vi "Multi-Record Acquisition with Queues.vi"() -> ()   [LabVIEW 2011]
uses:
  <vilib>/userDefined/High Color/nirio_resource_hc.ctl
  <vilib>/FPGAPlugInAG/PXIe-7965R/niLvFpga_Open_PXIe-7965R.vi
  <vilib>/rvi/interface/common/dynamic/niFpgaDynamicAddResources.vi
  <vilib>/FPGAPlugInAG/Dynamic/niLvFpga_Download_Dynamic.vi
  <vilib>/FPGAPlugInAG/Dynamic/niLvFpga_Run_Dynamic.vi
  <vilib>/Utility/error.llb/Error Cluster From Error Code.vi
  <vilib>/rvi/errors/niLvFpgaAdjustHostInterfaceError.vi
  <vilib>/FPGAPlugInAG/Dynamic/niLvFpga_Close_Dynamic.vi
  <vilib>/rvi/interface/nirviOpenFPGA/nirviOpenFPGA.xnode
  <userlib>/Fast OCT/Debug/Version 1/FPGA Bitfiles/Current/Acquire 2 channel data with DRAM (Multi-Record).lvbitx
  <vilib>/rvi/interface/nirviMethod/nirviMethod.xnode
  <vilib>/rvi/interface/nirviReadWriteControl/nirviReadWriteControl.xnode
  <vilib>/rvi/interface/nirviCloseFPGA/nirviCloseFPGA.xnode
  <userlib>/FlexRIO Host Library/FlexRIO Host Library (User).lvlib
  <vilib>/rvi/interface/Simulation/niFpgaSimulationCallBeginRW.vi
  NiFpgaLv.dll
panel:
  out "Consumer Stopped":bool
  out "Producer Stopped?":bool
  out "# elements in queue":i32
  out "Host FIFO Timed Out?":bool
  out "Buffer Timed Out?":bool
  out "Records Done":u32=500
  out "Elements Remaining":u32
  out "Iterations":i32=4
  in  "Display Raw Data?":bool=TRUE
  out "Channel Data":dbl[][](graph)
  out "Processing Time":u32=2246 format="%.0f ms"
  out "B-Scan Data":dbl[][](graph)
  in  "Device Name":T1="RIO0"
  in  "Stop":bool
  in  "Trigger Type":T2(ring)=enum."External Digital Trigger"
  in  "Record Count":u32=500
  in  "Pre Trig":u32=2
  in  "Post Trig":u32=1625
  out "error out":errorcluster
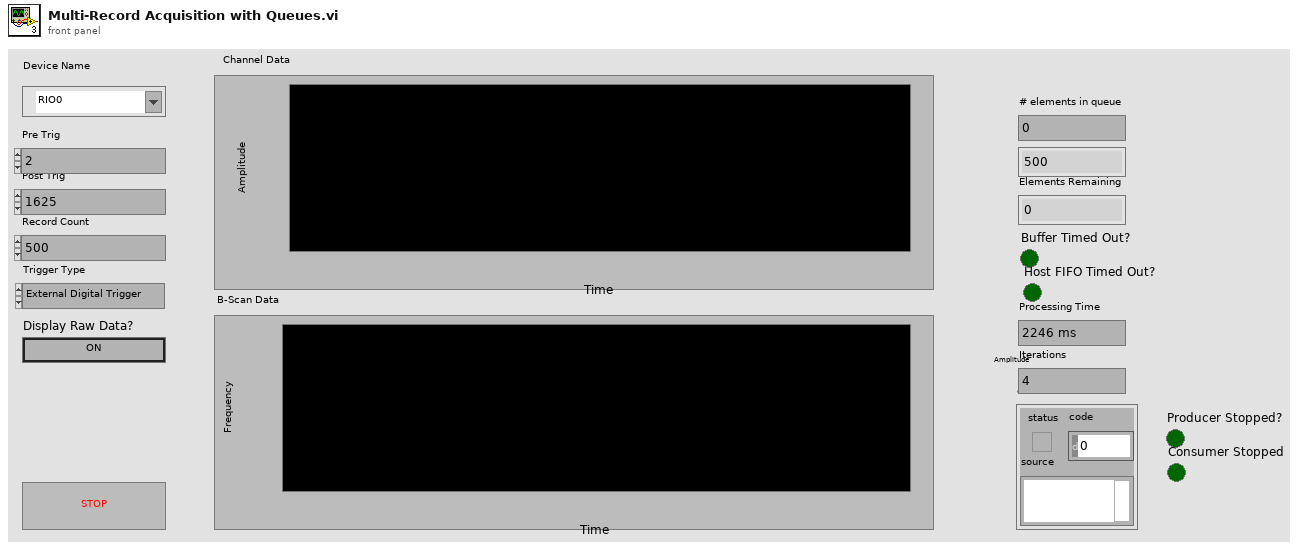
[diagram p1: front panel]
types:
  T1 = typedef "nirio_resource_hc.ctl" = tag
  T2 = enum8{"Immediate Trigger", "Software Trigger", "External Digital Trigger", "Analog Trigger"}
  T3 = cluster{"Load Record Parameters?":bool, "Pre Trigger Samples":u32, "Post Trigger Samples":u32, "Trigger Hold Off":u32, "Record Count":u32}
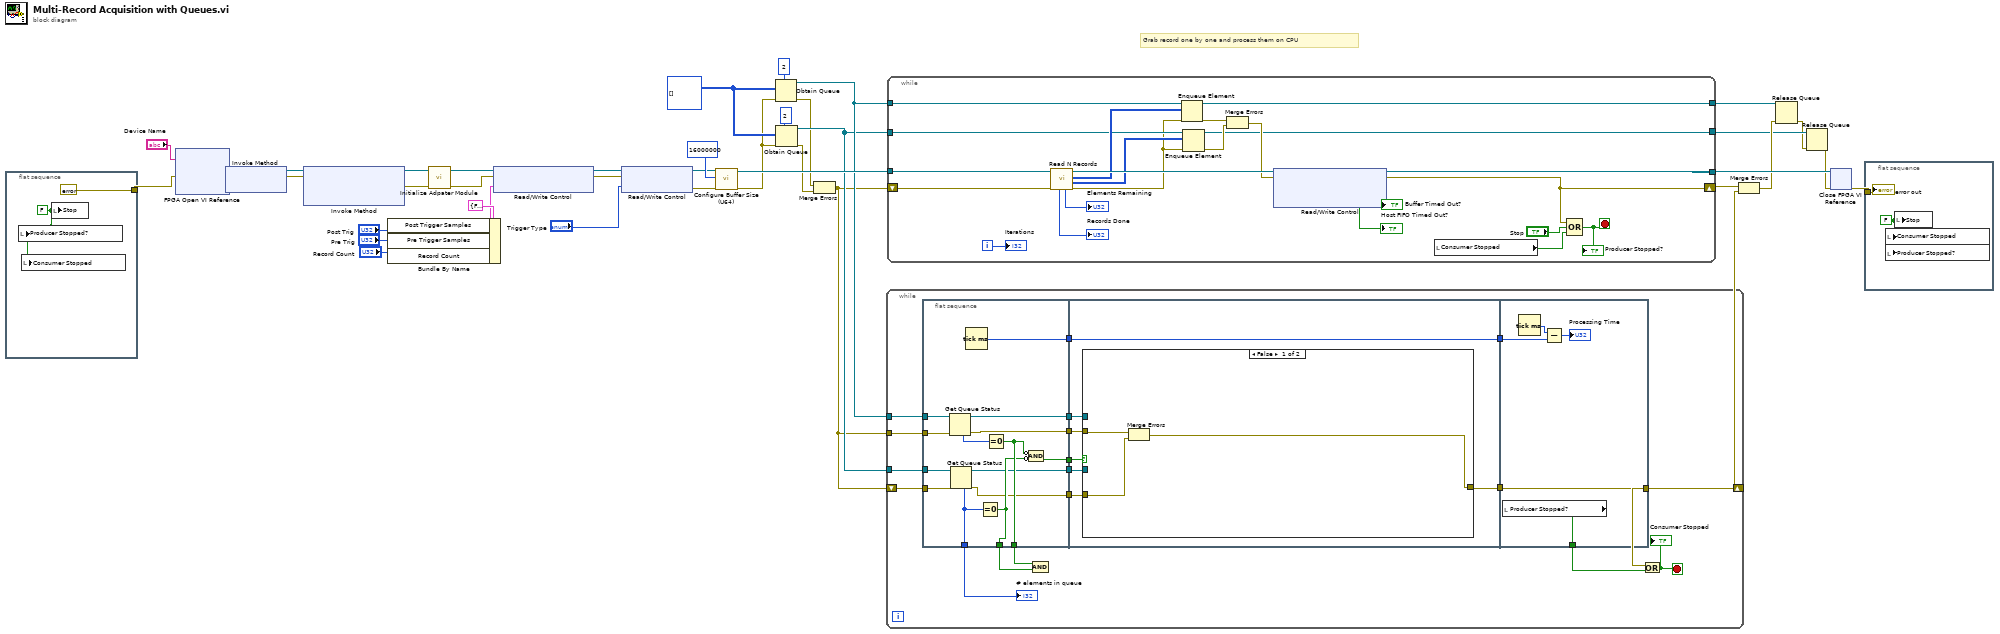
[diagram p0: block diagram]
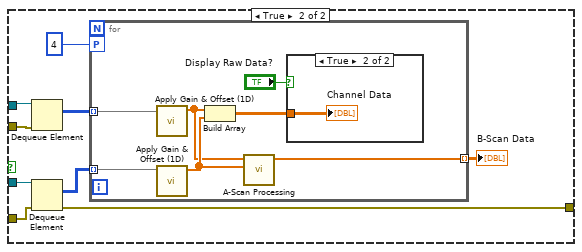
[diagram p2: hidden frame]
diagram:
  w16 = i16[][] [] ("Channel 1 Records")
  # "Grab record one by one and process them on CPU"
  n1 = flat-sequence {
    tunnel: [errorcluster {"status"=FALSE, "code"=0, "source"=""} ("error in")] -> w8
    frame #0 {
      w41 = FALSE ("Stop")
      n2 = local write "Producer Stopped?"(w41) -> ()
      n3 = local write "Consumer Stopped"(w41) -> ()
      n4 = local write "Stop"(w41) -> ()
    }
  }
  n5 = xnode "FPGA Open VI Reference"("error in"=w8, "resource name"="Device Name") -> ("FPGA VI Reference Out"=w22:refnum<k20>, "error out"=w23:errorcluster)
  n6 = xnode "Invoke Method"("FPGA VI Reference In"=w22, "error in"=w23) -> ("FPGA VI Reference Out"=w25:refnum<k20>, "error out"=w24:errorcluster)
  n7 = xnode "Invoke Method"("FPGA VI Reference In"=w25, "error in"=w24) -> ("FPGA VI Reference Out"=w36:refnum<k20>, "error out"=w35:errorcluster)  [unwired: 1 in]
  n8 = Bundle By Name(cluster=T3 {"Load Record Parameters?"=FALSE, "Pre Trigger Samples"=0, "Post Trigger Samples"=0, "Trigger Hold Off"=0, "Record Count"=0} ("Record Parameters"), "Post Trigger Samples"="Post Trig", "Pre Trigger Samples"="Pre Trig", "Record Count"="Record Count") -> (w20:T3)
  n9 = call <userlib>:"Initialize Adpater Module.vi"("error in"=w35, "FPGA VI Reference In"=w36) -> ("error out"=w38:errorcluster, "FPGA VI Reference Out"=w39:refnum<k20>)  [unwired: 7 in, 1 out]
  n10 = xnode "Read/Write Control"("FPGA VI Reference In"=w39, "error in"=w38, "Record Parameters"=w20) -> ("FPGA VI Reference Out"=w33:refnum<k20>, "error out"=w32:errorcluster)
  n11 = xnode "Read/Write Control"("FPGA VI Reference In"=w33, "error in"=w32, "Trigger Type"="Trigger Type") -> ("FPGA VI Reference Out"=w28:refnum<k20>, "error out"=w29:errorcluster)
  n12 = call <userlib>:"Configure Buffer Size (U64).vi"("error in"=w29, "Buffer Size"=u32 16000000, "FPGA VI Reference In"=w28) -> ("error out"=w14:errorcluster, "FPGA VI Reference Out"=w19:refnum<k20>)  [unwired: 7 in]
  n13 = Obtain Queue(max queue size (-1, unlimited)=2, element data type=w16, error in (no error)=w14) -> (queue out=w17:refnum<queue>, error out=w13:errorcluster)  [unwired: 2 in, 1 out]
  n14 = Obtain Queue(max queue size (-1, unlimited)=2, element data type=w16, error in (no error)=w14) -> (queue out=w15:refnum<queue>, error out=w12:errorcluster)  [unwired: 2 in, 1 out]
  n15 = Merge Errors(w13, w12) -> (w9:errorcluster)
  n16 = while {
    tunnel: w17 -> [w55]
    tunnel: w15 -> [w58]
    tunnel: w9 -> [w57]
    shift-right: [w44] -> w6
    shift-left: w9 -> [w56]
    stop <- w46 stop-if-true
    n17 = flat-sequence {
      tunnel: [w74] -> w60
      tunnel: w55 -> [w73]
      tunnel: w58 -> [w72]
      tunnel: w57 -> [w71]
      tunnel: w56 -> [w70]
      tunnel: [w69] -> w54
      tunnel: [w67] -> w53
      tunnel: [w66] -> w52
      tunnel: [w61] -> w51
      tunnel: [w65] -> w50
      tunnel: [w64] -> w49
      tunnel: [w63] -> w48
      tunnel: [w62] -> w47
      tunnel: w60 -> [w81]
      tunnel: [w81] -> w59
      tunnel: w54 -> [w80]
      tunnel: w50 -> [w79]
      tunnel: w49 -> [w78]
      tunnel: w48 -> [w77]
      tunnel: w47 -> [w76]
      tunnel: [w75] -> w45
      tunnel: w59 -> [w105]
      tunnel: w45 -> [w103]
      tunnel: [w103] -> w44
      tunnel: [w102] -> w43
      frame #0 {
        n18 = Get Queue Status(queue=w73, error in (no error)=w71) -> (queue out=w65:refnum<queue>, error out=w63:errorcluster, # elements in queue=w68:i32)  [unwired: 1 in, 5 out]
        n19 = Get Queue Status(queue=w72, error in (no error)=w70) -> (queue out=w64:refnum<queue>, error out=w62:errorcluster, # elements in queue=w61:i32)  [unwired: 1 in, 5 out]
        n20 = Tick Count (ms)() -> (millisecond timer value=w74:u32)
        n21 = Equal To 0?(x=w61) -> (x = 0?=w66:bool)
        n22 = Equal To 0?(x=w68) -> (x = 0?=w67:bool)
        n23 = Compound Arithmetic op=AND(invert w67, invert w66) -> (w69:bool)
      }
      frame #1 {
        n24 = case shown="False" w80 {
          tunnel: w79 -> [_ w91]
          tunnel: w78 -> [_ w88]
          tunnel: w77 -> [w84 w90]
          tunnel: w76 -> [w83 w87]
          tunnel: [w82 w85] -> w75
          frame False {
            n25 = Merge Errors(w84, w83) -> (w82:errorcluster)
          }
          frame True {
            n26 = Dequeue Element(queue=w91, error in (no error)=w90) -> (element=w89:i16[][])  [unwired: 1 in, 3 out]
            n27 = Dequeue Element(queue=w88, error in (no error)=w87) -> (element=w86:i16[][], error out=w85:errorcluster)  [unwired: 1 in, 2 out]
            n28 = for {
              tunnel: [w100] -> w93 mode=indexing
              workers-P: 4 -> [_]
              tunnel: w89 -> [w95] mode=indexing
              tunnel: w86 -> [w94] mode=indexing
              n29 = call <userlib>:"Apply Gain & Offset (1D).vi"("Raw Data"=w95) -> ("Scaled Data"=w97:dbl[])  [unwired: 10 in]
              n30 = call <userlib>:"Apply Gain & Offset (1D).vi"("Raw Data"=w94) -> ("Scaled Data"=w99:dbl[])  [unwired: 10 in]
              n31 = Build Array(w97, w99) -> (w98:dbl[][])
              n32 = call <userlib>:"A-Scan Processing.vi"("K-Clock"=w99, "OCT Signal"=w97) -> ("A-Scan"=w100:dbl[])  [unwired: 9 in]
              n33 = case shown="True" "Display Raw Data?" {
                tunnel: w98 -> [_ w101]
                frame False {
                }
                frame True {
                  "Channel Data" <- w101
                }
              }
            }
            "B-Scan Data" <- w93
          }
        }
      }
      frame #2 {
        n34 = local read "Producer Stopped?"() -> (w102:bool)
        n35 = Tick Count (ms)() -> (millisecond timer value=w106:u32)
        n36 = Subtract(x=w106, y=w105) -> (x-y=→"Processing Time":u32)
      }
    }
    n37 = Compound Arithmetic op=AND(w53, w52) -> ()  [unwired: 1 out]
    n38 = Or(x=w44, y=w43) -> (x .or. y?=w46:bool)
    "Consumer Stopped" <- w46
    "# elements in queue" <- w51
  }
  n39 = while {
    tunnel: w19 -> [w129]
    tunnel: [w121] -> w18
    shift-right: [w122] -> w7
    shift-left: w9 -> [w128]
    tunnel: w17 -> [w116]
    tunnel: w15 -> [w115]
    tunnel: [w110] -> w5
    tunnel: [w109] -> w3
    i -> [w126]
    stop <- w127 stop-if-true
    n40 = call <userlib>:"Read N Records.vi"("error in"=w128, "FPGA VI Reference In"=w129) -> ("error out"=w112:errorcluster, "Channel 1 Records"=w117:i16[][], "Channel 0 Records"=w118:i16[][], "FPGA VI Reference Out"=w123:refnum<k20>, "Elements Remaining"=→"Elements Remaining":u32, "Records Done"=→"Records Done":u32)  [unwired: 4 in]
    n41 = Enqueue Element(queue=w116, element=w118, error in (no error)=w112) -> (queue out=w110:refnum<queue>, error out=w114:errorcluster)  [unwired: 1 in, 1 out]
    n42 = Enqueue Element(queue=w115, element=w117, error in (no error)=w112) -> (queue out=w109:refnum<queue>, error out=w113:errorcluster)  [unwired: 1 in, 1 out]
    n43 = Merge Errors(w114, w113) -> (w111:errorcluster)
    n44 = xnode "Read/Write Control"("FPGA VI Reference In"=w123, "error in"=w111) -> ("FPGA VI Reference Out"=w121:refnum<k20>, "error out"=w122:errorcluster, "Buffer Timed Out?"=→"Buffer Timed Out?":bool, "Host FIFO Timed Out?"=→"Host FIFO Timed Out?":bool)
    n45 = local read "Consumer Stopped"() -> (w107:bool)
    n46 = Compound Arithmetic op=OR(w122, "Stop", w107) -> (w127:bool)
    "Producer Stopped?" <- w127
    "Iterations" <- w126
  }
  n47 = Merge Errors(w7, w6) -> (w4:errorcluster)
  n48 = Release Queue(queue=w5, error in (no error)=w4) -> (error out=w2:errorcluster)  [unwired: 1 in, 2 out]
  n49 = Release Queue(queue=w3, error in (no error)=w2) -> (error out=w1:errorcluster)  [unwired: 1 in, 2 out]
  n50 = xnode "Close FPGA VI Reference"("FPGA VI Reference In"=w18, "error in"=w1) -> ("error out"=w40:errorcluster)
  n51 = flat-sequence {
    tunnel: w40 -> [w131]
    frame #0 {
      w130 = FALSE ("Stop")
      n52 = local write "Consumer Stopped"(w130) -> ()
      n53 = local write "Producer Stopped?"(w130) -> ()
      n54 = local write "Stop"(w130) -> ()
      "error out" <- w131
    }
  }
